vi "BaslerFlyDetection.vi"(1 "image processing controls":T3={"Channel"=1, "Range"={"Lower value"=128.0, "Upper value"=255.0}, "downsampling"=1, "Operation"=0, "Interpolation Type"=0, "remove particle size"=2, "Single channel"=refnum, "Thresholded"=refnum, "raw image"=refnum, "subimage"=refnum} {"Interpolation Type" items=["Zero Order", "Bi-Linear", "Quadratic", "Cubic Spline"]; "Operation" items=["AutoM", "Close", "Dilate", "Erode", "Gradient", "Gradient out", "Gradient in", "Hit miss", "Open", "PClose", "POpen", "Thick", "Thin"]; "downsampling" min=1 max=24; "Range"."Upper value" format="%.2f"; "Range"."Lower value" format="%.2f"; "Channel" items=["Red", "Green", "Blue", "Hue", "Saturation", "Luminance", "Value", "Intensity"]}) -> (0 "image processing indicators":T2 {"Frame Rate" scale=0.0..35.0 scale format="%.1f"})   [LabVIEW 2012]
uses:
  <vilib>/vision/Image Controls.llb/IMAQ Image.ctl
  GlobalBaslerCamera.vi
  <vilib>/imath/engines/lvmath2/RunTimeEngine/ErrorHandling/NIMS_Finalize Error.vi
  <vilib>/imath/engines/lvmath2/RunTimeEngine/NodeEndStatement/NIMS_NodeEndStatement_Output.vi
  <instcachedir>/0/NIMS_NodeEndStatement_Output_53EC0D466D134D7ABD903AC30B43404B.lvgen/NIMS_NodeEndStatement_Output_53EC0D466D134D7ABD903AC30B43404B_004.vi
  <vilib>/imath/engines/lvmath2/RunTimeEngine/BuiltInFunctions/round/NIMS_round(DBL-M).vi
  <vilib>/imath/engines/lvmath2/RunTimeEngine/VariableToken/Read/NIMS_Get Elements - SorM(_) - Check.vi
  <instcachedir>/0/NIMS_Get Elements - SorM(_) - Check_8FDA2664A675493882C25203DD903B51.lvgen/NIMS_Get Elements - SorM(_) - Check_8FDA2664A675493882C25203DD903B51_000.vi
  <vilib>/imathl/engines/lvmath/Functions/Error Handling/Create Error.vi
  <vilib>/imath/engines/lvmath2/RunTimeEngine/ReplaceToken/NIMS_Replace - Check Linear.vi
  <instcachedir>/0/NIMS_Replace - Check Linear_44ABB4D6A819426DBDF25CCE6827BF1D.lvgen/NIMS_Replace - Check Linear_44ABB4D6A819426DBDF25CCE6827BF1D_001.vi
  <vilib>/imath/engines/lvmath2/RunTimeEngine/ReplaceToken/NIMS_Replace - Size Check _(_)=S.vi
  <instcachedir>/0/NIMS_Replace - Size Check _(_)=S_5AC8AA27B9694BB9828B57BCF666F597.lvgen/NIMS_Replace - Size Check _(_)=S_5AC8AA27B9694BB9828B57BCF666F597_000.vi
  <vilib>/imath/engines/lvmath2/RunTimeEngine/ReplaceToken/NIMS_Replace - V(S)=S.vi
  <instcachedir>/0/NIMS_Replace - V(S)=S_927EF1B21AA84780A9A306EC96B904EC.lvgen/NIMS_Replace - V(S)=S_927EF1B21AA84780A9A306EC96B904EC_000.vi
  <vilib>/imath/engines/lvmath2/RunTimeEngine/ErrorHandling/NIMS_Create Error From Enums.vi
  <instcachedir>/0/NIMS_Replace - Check Linear_44ABB4D6A819426DBDF25CCE6827BF1D.lvgen/NIMS_Replace - Check Linear_44ABB4D6A819426DBDF25CCE6827BF1D_010.vi
  <instcachedir>/0/NIMS_Replace - Size Check _(_)=S_5AC8AA27B9694BB9828B57BCF666F597.lvgen/NIMS_Replace - Size Check _(_)=S_5AC8AA27B9694BB9828B57BCF666F597_006.vi
  <instcachedir>/0/NIMS_Replace - V(S)=S_927EF1B21AA84780A9A306EC96B904EC.lvgen/NIMS_Replace - V(S)=S_927EF1B21AA84780A9A306EC96B904EC_004.vi
  <instcachedir>/0/NIMS_Replace - Check Linear_44ABB4D6A819426DBDF25CCE6827BF1D.lvgen/NIMS_Replace - Check Linear_44ABB4D6A819426DBDF25CCE6827BF1D_008.vi
  <instcachedir>/0/NIMS_Replace - Size Check _(_)=S_5AC8AA27B9694BB9828B57BCF666F597.lvgen/NIMS_Replace - Size Check _(_)=S_5AC8AA27B9694BB9828B57BCF666F597_007.vi
  <instcachedir>/0/NIMS_Replace - V(S)=S_927EF1B21AA84780A9A306EC96B904EC.lvgen/NIMS_Replace - V(S)=S_927EF1B21AA84780A9A306EC96B904EC_003.vi
  <vilib>/vision/driver/NI_Vision_Acquisition_Software.lvlib
  <vilib>/vision/NI_Vision_Development_Module.lvlib
  <resource>/objmgr/IMAQImage.rc
panel:
  out "image height":u32
  out "image width":u32
  in  "cropWidth 2":i32=600
  in  "cropWidth":i32=1200
  out "rectangle":i32[](array[numeric])
  out "resulting string":string
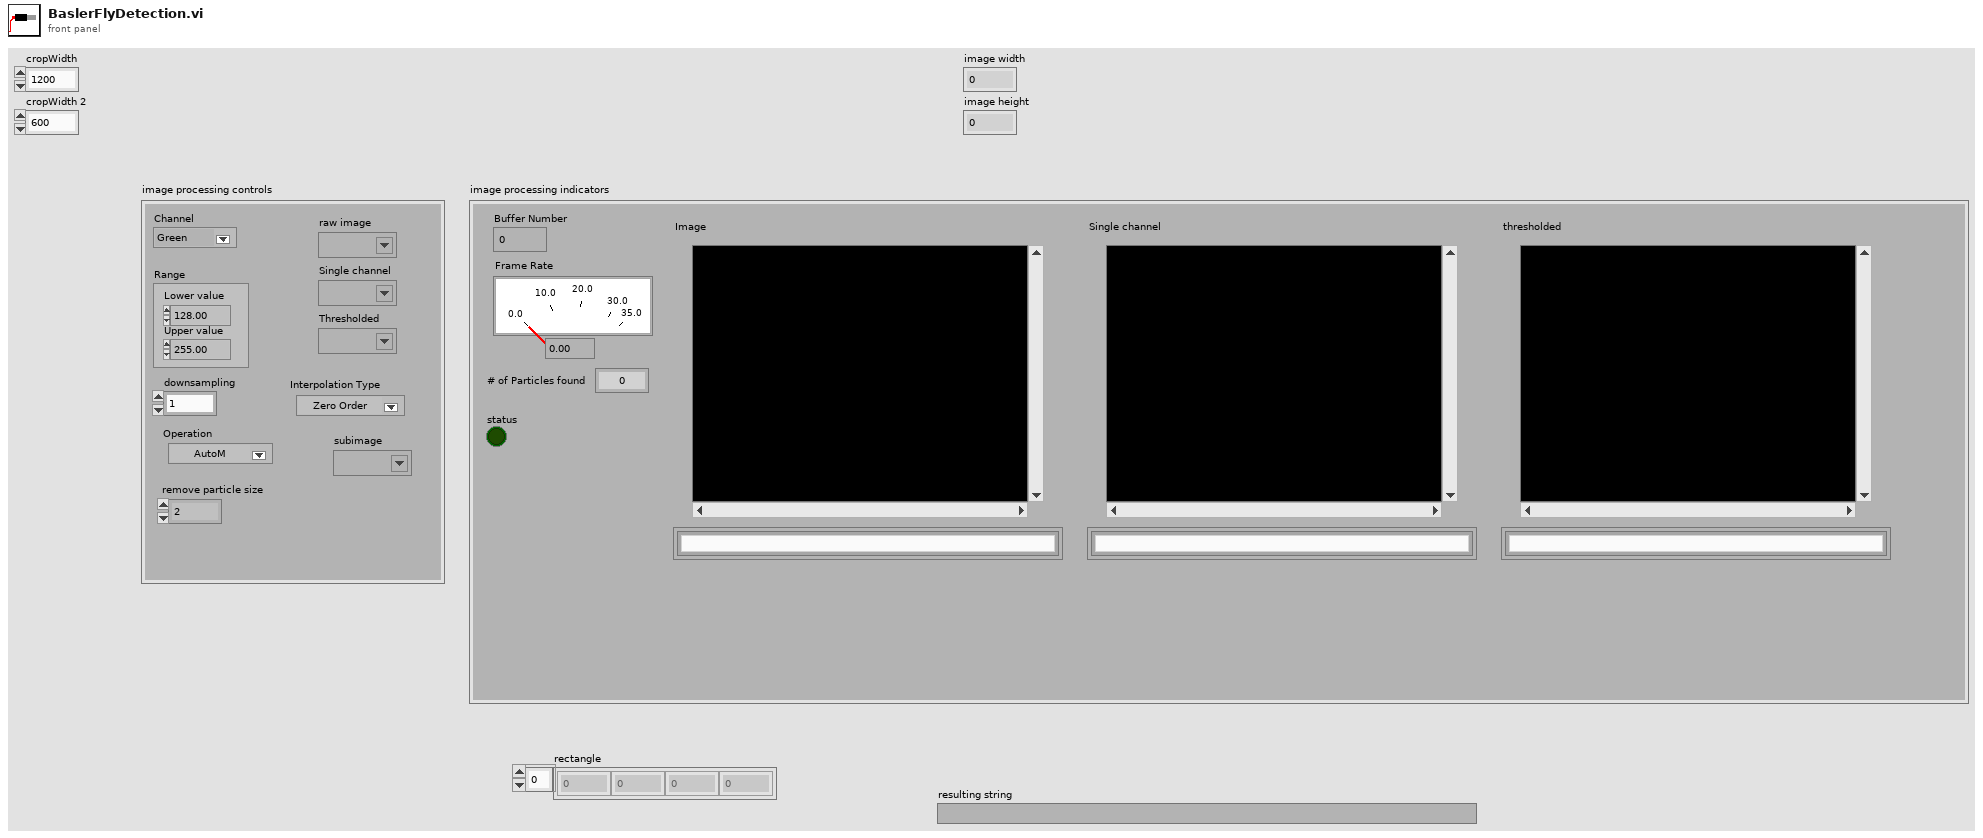
[diagram p1: front panel]
types:
  T1 = typedef "IMAQ Image.ctl" = refnum<image>
  T2 = cluster{"Buffer Number":u32, "Frame Rate":dbl, "# of Particles found":i32, "Image":T1, "Single channel":T1, "thresholded":T1, "status":bool}
  T3 = cluster{"Channel":i32, "Range":cluster{"Lower value":sgl, "Upper value":sgl}, "downsampling":u32, "Operation":u16, "Interpolation Type":u32, "remove particle size":i32, "Single channel":T1, "Thresholded":T1, "raw image":T1, "subimage":T1}
  T4 = typedef "IMAQdx.ctl" = refnum<k21>
  T5 = typedef "Particle Parameters" = i32
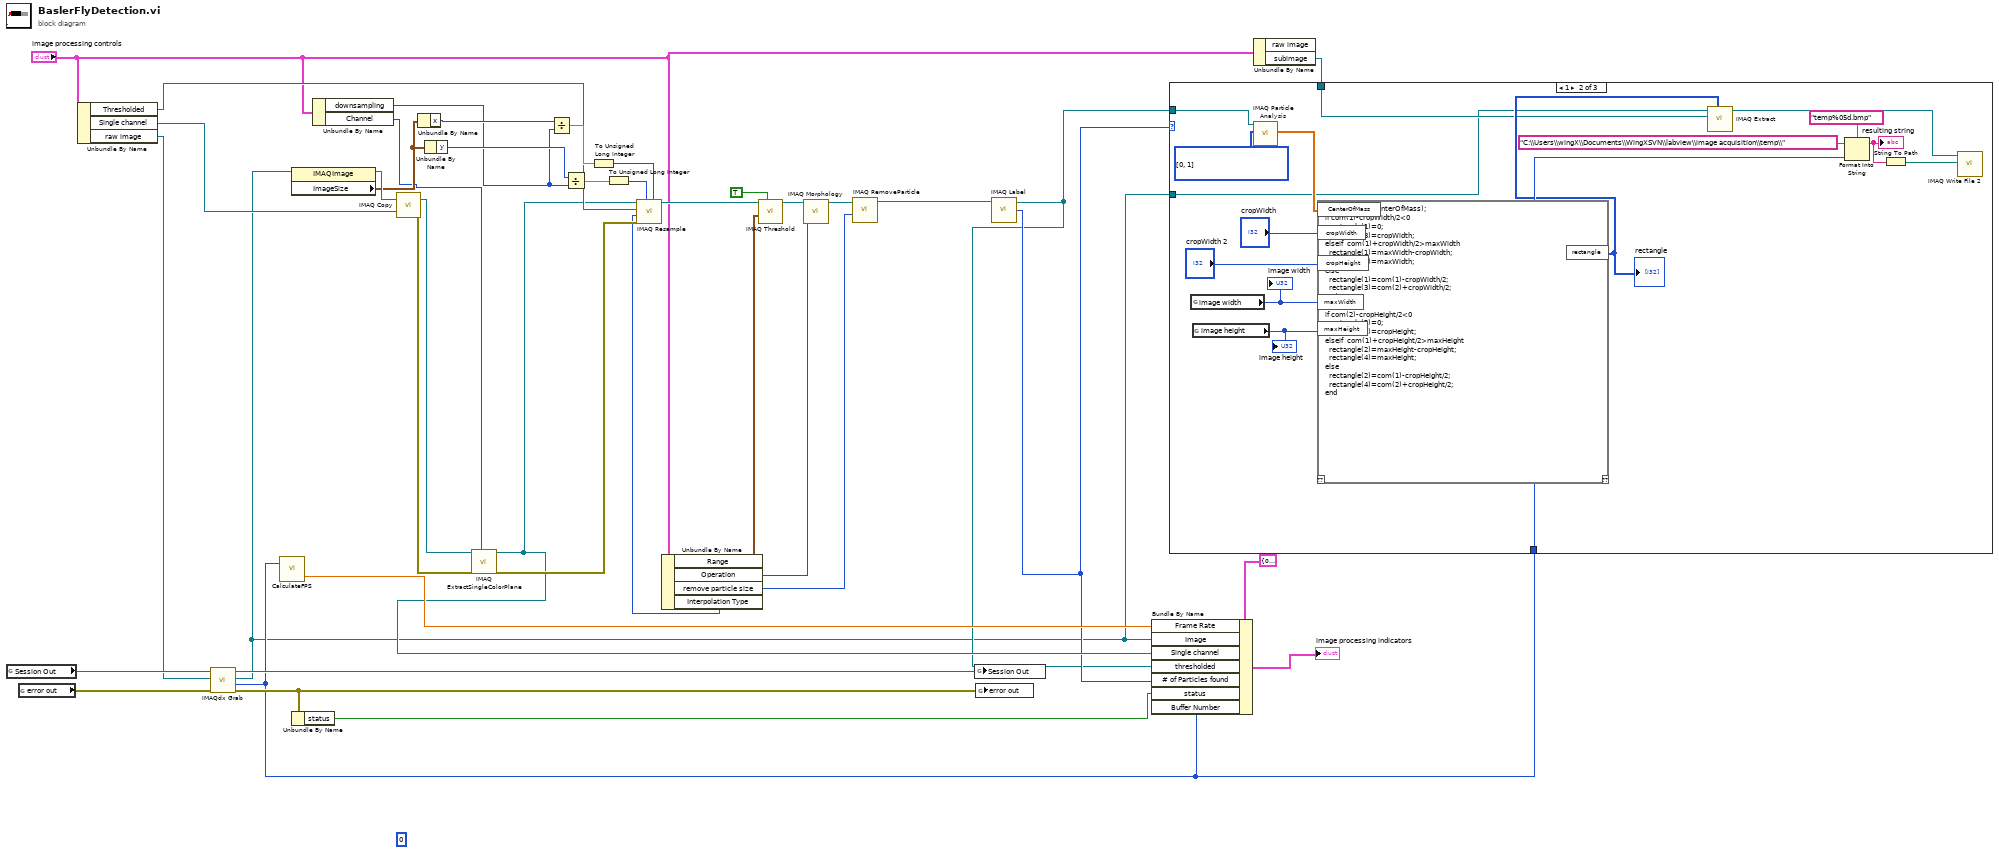
[diagram p0: block diagram]
diagram:
  (unwired) u32 0 ("Buffer Number Out")
  n1 = global read "GlobalBaslerCamera.vi" "Session Out"() -> (w40:T4)
  n2 = global read "GlobalBaslerCamera.vi" "error out"() -> (w39:errorcluster)
  n3 = Unbundle By Name("image processing controls") -> ("Thresholded"=w15:T1, "Single channel"=w14:T1, "raw image"=w13:T1)
  n4 = call <vilib>:"IMAQdx Grab.vi"("error in"=w39, "Image In"=w13, "Session In"=w40) -> ("error out"=w37:errorcluster, "Buffer Number Out"=w5:u32, "Image Out"=w1:T1, "Session Out"=w38:T4)  [unwired: 1 in, 4 out]
  n5 = call "CalculateFPS.vi"("buffer number"=w5) -> ("processed FPS"=w12:dbl)  [unwired: 1 in, 1 out]
  n6 = property class="IMAQImage"(reference=w1) -> (reference out=w27:T1, "ImageSize"=w24:cluster{"x":i32, "y":i32})  [unwired: 1 in, 1 out]
  n7 = Unbundle By Name(w37) -> ("status"=w8:bool)
  n8 = Unbundle By Name("image processing controls") -> ("downsampling"=w19:u32, "Channel"=w7:i32)
  n9 = call "IMAQ Copy"("Image Dst"=w14, "Image Src"=w27) -> ("error out"=w35:errorcluster, "Image Dst Out"=w36:T1)  [unwired: 4 in]
  n10 = Unbundle By Name(w24) -> ("x"=w26:i32)
  n11 = Unbundle By Name(w24) -> ("y"=w25:i32)
  n12 = call "IMAQ ExtractSingleColorPlane"("Color Plane"=w7, "error in (no error)"=w35, "Image Src"=w36) -> ("error out"=w34:errorcluster, "Image Dst Out"=w10:T1)  [unwired: 7 in]
  n13 = Divide(x=w26, y=w19) -> (x/y=w33:dbl)
  n14 = Divide(x=w25, y=w19) -> (x/y=w31:dbl)
  n15 = To Unsigned Long Integer(number=w33) -> (unsigned 32bit integer=w32:u32)
  n16 = To Unsigned Long Integer(number=w31) -> (unsigned 32bit integer=w30:u32)
  n17 = Unbundle By Name("image processing controls") -> ("Range"=w20:cluster{"Lower value":sgl, "Upper value":sgl}, "Operation"=w18:u16, "remove particle size"=w17:i32, "Interpolation Type"=w16:u32)
  n18 = call "IMAQ Resample"("X Resolution"=w32, "Y Resolution"=w30, "error in (no error)"=w34, "Interpolation Type"=w16, "Image Dst"=w15, "Image Src"=w10) -> ("Image Dst Out"=w29:T1)  [unwired: 4 in, 1 out]
  n19 = call "IMAQ Threshold"("Keep/Replace Value (Replace)"=TRUE, "Range"=w20, "Image Src"=w29) -> ("Image Dst Out"=w23:T1)  [unwired: 7 in, 1 out]
  n20 = call "IMAQ Morphology"("Operation"=w18, "Image Src"=w23) -> ("Image Dst Out"=w22:T1)  [unwired: 8 in, 1 out]
  n21 = call "IMAQ RemoveParticle"("Number of Erosion"=w17, "Image Src"=w22) -> ("Image Dst Out"=w21:T1)  [unwired: 8 in, 1 out]
  n22 = global write "GlobalBaslerCamera.vi" "Session Out"(w38) -> ()
  n23 = global write "GlobalBaslerCamera.vi" "error out"(w37) -> ()
  n24 = call "IMAQ Label"("Image Src"=w21) -> ("Number of Particles"=w6:i32, "Image Dst Out"=w4:T1)  [unwired: 3 in, 1 out]
  n25 = Bundle By Name(cluster=T2 {"Buffer Number"=0, "Frame Rate"=20.58254552990705, "# of Particles found"=3, "Image"="Vision Acq Image 47498962Untitled 1:Instance:0<Not A Path>", "Single channel"="single", "thresholded"="thresholded", "status"=TRUE} ("image processing indicators"), "Frame Rate"=w12, "Image"=w1, "Single channel"=w10, "thresholded"=w4, "# of Particles found"=w6, "status"=w8, "Buffer Number"=w5) -> (→"image processing indicators":T2)
  n26 = Unbundle By Name("image processing controls") -> ("subimage"=w2:T1)  [unwired: 1 out]
  n27 = case shown="1" w6 {
    tunnel: w5 -> [_ w52 _]
    tunnel: w4 -> [_ w45 _]
    tunnel: w2 -> [_ w42 _]
    tunnel: w1 -> [_ w41 _]
    frame 0 {
    }
    frame 1 {
      w51 = T5[] [0, 1] items=["Center of Mass X", "Center of Mass Y", "First Pixel X", "First Pixel Y", "Bounding Rect Left", "Bounding Rect Top", "Bounding Rect Right", "Bounding Rect Bottom", "Max Feret Diameter Start X", "Max Feret Diameter Start Y", "Max Feret Diameter End X", "Max Feret Diameter End Y", "Max Horiz. Segment Length Left", "Max Horiz. Segment Length Right", "Max Horiz. Segment Length Row", "-", "Bounding Rect Width", "Bounding Rect Height", "Bounding Rect Diagonal", "Perimeter", "Convex Hull Perimeter", "Holes' Perimeter", "Max Feret Diameter", "Equivalent Ellipse Major Axis", "Equivalent Ellipse Minor Axis", "Equivalent Ellipse Minor Axis (Feret)", "Equivalent Rect Long Side", "Equivalent Rect Short Side", "Equivalent Rect Diagonal", "Equivalent Rect Short Side (Feret)", "Average Horiz. Segment Length", "Average Vert. Segment Length", "Hydraulic Radius", "Waddel Disk Diameter", "-", "Area", "Holes' Area", "Particle & Holes' Area", "Convex Hull Area", "Image Area", "-", "Number of Holes", "Number of Horiz. Segments", "Number of Vert. Segments", "-", "Orientation", "Max Feret Diameter Orientation", "-", "% Area/Image Area", "% Area/(Particle & Holes' Area)", "Ratio of Equivalent Ellipse Axes", "Ratio of Equivalent Rect Sides", "-", "Elongation Factor", "Compactness Factor", "Heywood Circularity Factor", "Type Factor", "-", "Sum X", "Sum Y", "Sum XX", "Sum XY", "Sum YY", "Sum XXX", "Sum XXY", "Sum XYY", "Sum YYY", "-", "Moment of Inertia XX", "Moment of Inertia XY", "Moment of Inertia YY", "Moment of Inertia XXX", "Moment of Inertia XXY", "Moment of Inertia XYY", "Moment of Inertia YYY", "Norm. Moment of Inertia XX", "Norm. Moment of Inertia XY", "Norm. Moment of Inertia YY", "Norm. Moment of Inertia XXX", "Norm. Moment of Inertia XXY", "Norm. Moment of Inertia XYY", "Norm. Moment of Inertia YYY", "Hu Moment 1", "Hu Moment 2", "Hu Moment 3", "Hu Moment 4", "Hu Moment 5", "Hu Moment 6", "Hu Moment 7"] ("Pixel Measurements")
      n28 = global read "GlobalBaslerCamera.vi" "image width"() -> (w48:u32)
      "image width" <- w48
      n29 = global read "GlobalBaslerCamera.vi" "image height"() -> (w47:u32)
      "image height" <- w47
      n30 = call "IMAQ Particle Analysis"("Pixel Measurements"=w51, "Image"=w45) -> ("Particle Measurements (Pixels)"=w50:dbl[][])  [unwired: 3 in, 6 out]
      n31 = mathscript code="com = round(CenterOfMass);\nif com(1)-cropWidth/2<0\n  rectangle(1)=0;\n  rectangle(3)=cropWidth;\nelseif  com(1)+cropWidth/2>maxWidth\n  rectangle(1)=maxWidth-cropWidth;\n  rectangle(3)=maxWidth;\nelse\n  rectangle(1)=com(1)-cropWidth/2;\n  rectangle(3)=com(2)+cropWidth/2;\nend\n\nif com(2)-cropHeight/2<0\n  rectangle(2)=0;\n  rectangle(4)=cropHeight;\nelseif  com(1)+cropHeight/2>maxHeight\n  rectangle(2)=maxHeight-cropHeight;\n  rectangle(4)=maxHeight;\nelse\n  rectangle(2)=com(1)-cropHeight/2;\n  rectangle(4)=com(2)+cropHeight/2;\nend"("CenterOfMass"=w50, "cropWidth"="cropWidth", "maxWidth"=w48, "maxHeight"=w47, "cropHeight"="cropWidth 2") -> ("rectangle"=w43:i32[])  [unwired: 1 in, 1 out]
      "rectangle" <- w43
      n32 = call "IMAQ Extract"("Optional Rectangle"=w43, "Image Dst"=w42, "Image Src"=w41) -> ("Image Dst Out"=w44:T1)  [unwired: 7 in, 1 out]
      n33 = Format Into String(format string="temp%05d.bmp", initial string="C:\\Users\\wingX\\Documents\\WingXSVN\\labview\\image acquisition\\temp\\", w52) -> (resulting string=w54:string)  [unwired: 1 in, 1 out]
      "resulting string" <- w54
      n34 = String To Path(string=w54) -> (path=w53:path)
      n35 = call-poly "IMAQ Write File 2"("File Path"=w53, "Image"=w44) -> ()  [unwired: 8 in, 2 out]
    }
    frame 2, Default {
    }
  }
